vi "TLB Native Dynamic Events ver 0.26c.vi"() -> ()   [LabVIEW 2018] (continued)
                  tunnel: [w1148 w1154] -> w1144
                  tunnel: w1136 -> [w1146 w1152]
                  frame False {
                    n432 = for {
                      tunnel: string[] ["START TIMER", "OPEN CLAW", ""] ("element") -> [w1149] mode=indexing
                      shift-right: [w1151] -> w1148
                      shift-left: w1146 -> [w1150]
                      n433 = Enqueue Element(queue=w1150, element=w1149) -> (queue out=w1151:refnum<queue>)  [unwired: 2 in, 2 out]
                    }
                  }
                  frame True {
                    n434 = for {
                      shift-right: [w1156] -> w1154
                      shift-left: w1152 -> [w1157]
                      tunnel: string[] ["CAM CLOSE", "", ""] -> [w1155] mode=indexing
                      n435 = Enqueue Element(queue=w1157, element=w1155) -> (queue out=w1156:refnum<queue>)  [unwired: 2 in, 2 out]
                    }
                  }
                }
                n436 = Or(x=w1135, y=w1140) -> (x .or. y?=w1142:bool)
                n437 = Select(t=State_Type_Definitions,_for_0.26g_versions_and_later_2."True Stop" ("Enum"), s=w1140, f=State_Type_Definitions,_for_0.26g_versions_and_later_2."True Stop" ("Enum")) -> (s? t:f=w1137:T18)
                n438 = Select(t=w1137, s=w1142, f=State_Type_Definitions,_for_0.26g_versions_and_later_2."Task 5D" ("Enum")) -> (s? t:f=w1141:T18)
              }
              frame "Exit" {
                n439 = for {
                  shift-right: [w1164] -> w1161
                  shift-left: w1158 -> [w1165]
                  tunnel: string[] ["STOP", "RESET ENCODERS", "RESET YAW", "ARDUINO MODE 0"] -> [w1163] mode=indexing
                  n440 = Enqueue Element(queue=w1165, element=w1163) -> (queue out=w1164:refnum<queue>)  [unwired: 2 in, 2 out]
                }
              }
            }
          }
          frame 20 {
            # ">>> yStepper command>>>"
            n441 = Dequeue Element(queue=w1179, timeout in ms (-1)=w1180, error in (no error)=w1181) -> (element=w1183:T10)  [unwired: 3 out]
            n442 = formula code="if (pos < 100)\ny = 41;\n\nelse if (pos >= 100 && pos <= 140)\ny = 30;\n\nelse if (pos >= 141 && pos <= 170)\ny = 25;\n\nelse if (pos >= 171 &&pos <= 180) \ny = 20;\n\nelse if (pos >= 181&& pos <= 200)\ny = 15;\n\nelse if (pos >= 201 && pos <= 230)\ny = 10;\n\nelse if (pos >= 231 && pos <= 320)\ny = 8;\n\nelse if (pos > 320)\ny = 0;"("pos"=w1171) -> ("y"=w1174:dbl)
            n443 = To Unsigned Byte Integer(number=w1174) -> (unsigned 8bit integer=w1169:u8)
            n444 = Equal?(x=w1170, y=w1169) -> (x = y?=w1168:bool)
            n445 = case shown="\"Start Task 1\", Default" w1183 {
              tunnel: [w1190 State_Type_Definitions,_for_0.26g_versions_and_later_2."True Stop" ("Enum")] -> w1177
              tunnel: [w1193 w1210] -> w1175
              tunnel: [State_Type_Definitions,_for_0.26g_versions_and_later_2."Idle" ("Enum") State_Type_Definitions,_for_0.26g_versions_and_later_2."Shutdown" ("Enum")] -> w1176
              tunnel: w1182 -> [w1189 _]
              tunnel: w1178 -> [w1185 w1207]
              tunnel: w1168 -> [w1184 _]
              frame "Start Task 1", Default {
                # ">> T: Breaks out of state loop; F: Stays in loop>>"
                # ">> Manual override >>"
                # ">> Checks if time is up>>"
                # "Stays in Task 5D until the object is detected"
                # "T: Go back to idle, F: Continue with task\""
                # ">> Manual override >>"
                n446 = case shown="False" w1184 {
                  tunnel: [w1197 w1203] -> w1193
                  tunnel: w1185 -> [w1195 w1201]
                  frame False {
                    n447 = for {
                      tunnel: string[] ["READ STEPPER VALUES", "Y STEPPER CONTROL", ""] ("element") -> [w1198] mode=indexing
                      shift-right: [w1200] -> w1197
                      shift-left: w1195 -> [w1199]
                      n448 = Enqueue Element(queue=w1199, element=w1198) -> (queue out=w1200:refnum<queue>)  [unwired: 2 in, 2 out]
                    }
                  }
                  frame True {
                    n449 = for {
                      shift-right: [w1205] -> w1203
                      shift-left: w1201 -> [w1206]
                      tunnel: string[] ["CAM CLOSE", "DISPOSE BUFFERS", ""] -> [w1204] mode=indexing
                      n450 = Enqueue Element(queue=w1206, element=w1204) -> (queue out=w1205:refnum<queue>)  [unwired: 2 in, 2 out]
                    }
                  }
                }
                n451 = Or(x=w1184, y=w1189) -> (x .or. y?=w1191:bool)
                n452 = Select(t=State_Type_Definitions,_for_0.26g_versions_and_later_2."True Stop" ("Enum"), s=w1189, f=State_Type_Definitions,_for_0.26g_versions_and_later_2."Task 5F: ARM GRAB HEIGHT" ("Enum")) -> (s? t:f=w1186:T18)
                n453 = Select(t=w1186, s=w1191, f=State_Type_Definitions,_for_0.26g_versions_and_later_2."Task 5E: POSITION ARM" ("Enum")) -> (s? t:f=w1190:T18)
              }
              frame "Exit" {
                n454 = for {
                  shift-right: [w1213] -> w1210
                  shift-left: w1207 -> [w1214]
                  tunnel: string[] ["STOP", "RESET ENCODERS", "RESET YAW", "ARDUINO MODE 0"] -> [w1212] mode=indexing
                  n455 = Enqueue Element(queue=w1214, element=w1212) -> (queue out=w1213:refnum<queue>)  [unwired: 2 in, 2 out]
                }
              }
            }
            n456 = Bundle By Name(cluster=w1173, "yStepper desired"=w1169) -> (w1172:T20)
          }
          frame 21 {
            # ">>> Motor control cluster >>>"
            # ">>> yStepper command>>>"
            # ">> Manual override >>"
            n457 = Dequeue Element(queue=w1225, timeout in ms (-1)=w1224, error in (no error)=w1226) -> (element=w1223:T10)  [unwired: 3 out]
            n458 = Equal?(x=w1222, y=u8 1) -> (x = y?=w1220:bool)
            n459 = case shown="\"Start Task 1\", Default" w1223 {
              tunnel: [w1236 State_Type_Definitions,_for_0.26g_versions_and_later_2."True Stop" ("Enum")] -> w1227
              tunnel: [w1239 w1256] -> w1228
              tunnel: [State_Type_Definitions,_for_0.26g_versions_and_later_2."Idle" ("Enum") State_Type_Definitions,_for_0.26g_versions_and_later_2."Shutdown" ("Enum")] -> w1229
              tunnel: w1220 -> [w1235 _]
              tunnel: w1219 -> [w1234 _]
              tunnel: w1218 -> [w1230 w1253]
              frame "Start Task 1", Default {
                # "Stays in Task 5F until stepper reaches desired \nheight"
                # "T: Go back to idle, F: Continue with task\""
                # ">> Manual override >>"
                n460 = case shown="True" w1235 {
                  tunnel: [w1243 w1249] -> w1239
                  tunnel: w1230 -> [w1241 w1247]
                  frame False {
                    n461 = for {
                      tunnel: string[] ["Z STEPPER GRAB HEIGHT", "READ STEPPER VALUES"] ("element") -> [w1244] mode=indexing
                      shift-right: [w1246] -> w1243
                      shift-left: w1241 -> [w1245]
                      n462 = Enqueue Element(queue=w1245, element=w1244) -> (queue out=w1246:refnum<queue>)  [unwired: 2 in, 2 out]
                    }
                  }
                  frame True {
                    n463 = for {
                      shift-right: [w1251] -> w1249
                      shift-left: w1247 -> [w1252]
                      tunnel: string[] ["SET TIMER 5", "CLOSE CLAW", ""] -> [w1250] mode=indexing
                      n464 = Enqueue Element(queue=w1252, element=w1250) -> (queue out=w1251:refnum<queue>)  [unwired: 2 in, 2 out]
                    }
                  }
                }
                n465 = Or(x=w1235, y=w1234) -> (x .or. y?=w1237:bool)
                n466 = Select(t=State_Type_Definitions,_for_0.26g_versions_and_later_2."True Stop" ("Enum"), s=w1234, f=State_Type_Definitions,_for_0.26g_versions_and_later_2."Task 5G: CLOSE CLAW" ("Enum")) -> (s? t:f=w1231:T18)
                n467 = Select(t=w1231, s=w1237, f=State_Type_Definitions,_for_0.26g_versions_and_later_2."Task 5F: ARM GRAB HEIGHT" ("Enum")) -> (s? t:f=w1236:T18)
              }
              frame "Exit" {
                n468 = for {
                  shift-right: [w1259] -> w1256
                  shift-left: w1253 -> [w1260]
                  tunnel: string[] ["STOP", "RESET ENCODERS", "RESET YAW", "ARDUINO MODE 0"] -> [w1258] mode=indexing
                  n469 = Enqueue Element(queue=w1260, element=w1258) -> (queue out=w1259:refnum<queue>)  [unwired: 2 in, 2 out]
                }
              }
            }
          }
          frame 22 {
            # ">>> yStepper command>>>"
            # ">> Manual override >>"
            n470 = Dequeue Element(queue=w1271, timeout in ms (-1)=w1270, error in (no error)=w1269) -> (element=w1268:T10)  [unwired: 3 out]
            n471 = case shown="\"Start Task 1\", Default" w1268 {
              tunnel: [w1280 State_Type_Definitions,_for_0.26g_versions_and_later_2."True Stop" ("Enum")] -> w1273
              tunnel: [w1283 w1300] -> w1266
              tunnel: [State_Type_Definitions,_for_0.26g_versions_and_later_2."Idle" ("Enum") State_Type_Definitions,_for_0.26g_versions_and_later_2."Shutdown" ("Enum")] -> w1265
              tunnel: w1267 -> [w1274 _]
              tunnel: w1272 -> [w1279 w1297]
              tunnel: w1263 -> [w1278 _]
              frame "Start Task 1", Default {
                # ">> Is time up? >>"
                # "Determines if object is in range to pick up"
                # ">> Manual override >>"
                n472 = case shown="True" w1278 {
                  tunnel: [w1287 w1293] -> w1283
                  tunnel: w1279 -> [w1285 w1291]
                  frame False {
                    n473 = for {
                      tunnel: string[] ["CLOSE CLAW", "START TIMER"] ("element") -> [w1288] mode=indexing
                      shift-right: [w1290] -> w1287
                      shift-left: w1285 -> [w1289]
                      n474 = Enqueue Element(queue=w1289, element=w1288) -> (queue out=w1290:refnum<queue>)  [unwired: 2 in, 2 out]
                    }
                  }
                  frame True {
                    n475 = for {
                      shift-right: [w1295] -> w1293
                      shift-left: w1291 -> [w1296]
                      tunnel: string[] ["READ STEPPER VALUES", "", ""] -> [w1294] mode=indexing
                      n476 = Enqueue Element(queue=w1296, element=w1294) -> (queue out=w1295:refnum<queue>)  [unwired: 2 in, 2 out]
                    }
                  }
                }
                n477 = Or(x=w1278, y=w1274) -> (x .or. y?=w1281:bool)
                n478 = Select(t=State_Type_Definitions,_for_0.26g_versions_and_later_2."True Stop" ("Enum"), s=w1274, f=State_Type_Definitions,_for_0.26g_versions_and_later_2."Task 5H: RAISE ARM" ("Enum")) -> (s? t:f=w1276:T18)
                n479 = Select(t=w1276, s=w1281, f=State_Type_Definitions,_for_0.26g_versions_and_later_2."Task 5G: CLOSE CLAW" ("Enum")) -> (s? t:f=w1280:T18)
              }
              frame "Exit" {
                n480 = for {
                  shift-right: [w1303] -> w1300
                  shift-left: w1297 -> [w1304]
                  tunnel: string[] ["STOP", "RESET ENCODERS", "RESET YAW", "ARDUINO MODE 0"] -> [w1302] mode=indexing
                  n481 = Enqueue Element(queue=w1304, element=w1302) -> (queue out=w1303:refnum<queue>)  [unwired: 2 in, 2 out]
                }
              }
            }
          }
          frame 23 {
            # ">>> yStepper command>>>"
            # ">> Manual override >>"
            n482 = Dequeue Element(queue=w1315, timeout in ms (-1)=w1314, error in (no error)=w1316) -> (element=w1313:T10)  [unwired: 3 out]
            n483 = Equal?(x=w1312, y=u8 60) -> (x = y?=w1310:bool)
            n484 = case shown="\"Start Task 1\", Default" w1313 {
              tunnel: [w1326 State_Type_Definitions,_for_0.26g_versions_and_later_2."True Stop" ("Enum")] -> w1317
              tunnel: [w1329 w1346] -> w1318
              tunnel: [State_Type_Definitions,_for_0.26g_versions_and_later_2."Idle" ("Enum") State_Type_Definitions,_for_0.26g_versions_and_later_2."Shutdown" ("Enum")] -> w1319
              tunnel: w1310 -> [w1325 _]
              tunnel: w1309 -> [w1324 _]
              tunnel: w1308 -> [w1320 w1343]
              frame "Start Task 1", Default {
                # "Stays in Task 5_A until stepper reaches desired \nheight"
                # "T: Go back to idle, F: Continue with task\""
                # ">> Manual override >>"
                n485 = case shown="False" w1325 {
                  tunnel: [w1333 w1339] -> w1329
                  tunnel: w1320 -> [w1331 w1337]
                  frame False {
                    n486 = for {
                      tunnel: string[] ["Z STEPPER CAM HEIGHT", "READ STEPPER VALUES"] ("element") -> [w1334] mode=indexing
                      shift-right: [w1336] -> w1333
                      shift-left: w1331 -> [w1335]
                      n487 = Enqueue Element(queue=w1335, element=w1334) -> (queue out=w1336:refnum<queue>)  [unwired: 2 in, 2 out]
                    }
                  }
                  frame True {
                    n488 = for {
                      shift-right: [w1341] -> w1339
                      shift-left: w1337 -> [w1342]
                      tunnel: string[] ["ARDUINO - ULTRASONIC", "READ ULTRASONIC", ""] -> [w1340] mode=indexing
                      n489 = Enqueue Element(queue=w1342, element=w1340) -> (queue out=w1341:refnum<queue>)  [unwired: 2 in, 2 out]
                    }
                  }
                }
                n490 = Or(x=w1325, y=w1324) -> (x .or. y?=w1327:bool)
                n491 = Select(t=State_Type_Definitions,_for_0.26g_versions_and_later_2."True Stop" ("Enum"), s=w1324, f=State_Type_Definitions,_for_0.26g_versions_and_later_2."True Stop" ("Enum")) -> (s? t:f=w1321:T18)
                n492 = Select(t=w1321, s=w1327, f=State_Type_Definitions,_for_0.26g_versions_and_later_2."Task 5H: RAISE ARM" ("Enum")) -> (s? t:f=w1326:T18)
              }
              frame "Exit" {
                n493 = for {
                  shift-right: [w1349] -> w1346
                  shift-left: w1343 -> [w1350]
                  tunnel: string[] ["STOP", "RESET ENCODERS", "RESET YAW", "ARDUINO MODE 0"] -> [w1348] mode=indexing
                  n494 = Enqueue Element(queue=w1350, element=w1348) -> (queue out=w1349:refnum<queue>)  [unwired: 2 in, 2 out]
                }
              }
            }
          }
          frame 24 {
            # ">>> yStepper command>>>"
            n495 = Dequeue Element(queue=w1360, timeout in ms (-1)=w1359, error in (no error)=w1358) -> (element=w1365:T10)  [unwired: 3 out]
            n496 = Equal?(x=w1356, y=u8 60) -> (x = y?=w1355:bool)
            n497 = case shown="\"Start Task 1\", Default" w1365 {
              tunnel: [w1372 State_Type_Definitions,_for_0.26g_versions_and_later_2."True Stop" ("Enum")] -> w1363
              tunnel: [w1371 w1389] -> w1362
              tunnel: [State_Type_Definitions,_for_0.26g_versions_and_later_2."Idle" ("Enum") State_Type_Definitions,_for_0.26g_versions_and_later_2."Shutdown" ("Enum")] -> w1364
              tunnel: w1361 -> [w1367 _]
              tunnel: w1357 -> [w1369 _]
              tunnel: w1355 -> [w1366 _]
              frame "Start Task 1", Default {
                n498 = case shown="False" w1366 {
                  tunnel: [w1377 w1383] -> w1371
                  tunnel: w1369 -> [w1375 w1381]
                  frame False {
                    n499 = for {
                      tunnel: string[] ["Z STEPPER CAM HEIGHT", "READ STEPPER VALUES"] ("element") -> [w1378] mode=indexing
                      shift-right: [w1380] -> w1377
                      shift-left: w1375 -> [w1379]
                      n500 = Enqueue Element(queue=w1379, element=w1378) -> (queue out=w1380:refnum<queue>)  [unwired: 2 in, 2 out]
                    }
                  }
                  frame True {
                    n501 = for {
                      shift-right: [w1385] -> w1383
                      shift-left: w1381 -> [w1386]
                      tunnel: string[] ["CAM ACQ", "OPEN LOG CAM"] -> [w1384] mode=indexing
                      n502 = Enqueue Element(queue=w1386, element=w1384) -> (queue out=w1385:refnum<queue>)  [unwired: 2 in, 2 out]
                    }
                  }
                }
                n503 = Or(x=w1366, y=w1367) -> (x .or. y?=w1368:bool)
                n504 = Select(t=State_Type_Definitions,_for_0.26g_versions_and_later_2."Task 6_B" ("Enum"), s=w1368, f=State_Type_Definitions,_for_0.26g_versions_and_later_2."Task 6_A" ("Enum")) -> (s? t:f=w1372:T18)
              }
              frame "Exit" {
                n505 = for {
                  shift-right: [w1392] -> w1389
                  shift-left: _ -> [w1393]
                  tunnel: string[] ["STOP", "RESET ENCODERS", "RESET YAW", "ARDUINO MODE 0"] -> [w1391] mode=indexing
                  n506 = Enqueue Element(queue=w1393, element=w1391) -> (queue out=w1392:refnum<queue>)  [unwired: 2 in, 2 out]
                }
              }
            }
          }
          frame 25 {
            # ">>> yStepper command>>>"
            n507 = Dequeue Element(queue=w1405, timeout in ms (-1)=w1403, error in (no error)=w1404) -> (element=w1402:T10)  [unwired: 3 out]
            n508 = case shown="\"Start Task 1\", Default" w1402 {
              tunnel: [w1412 State_Type_Definitions,_for_0.26g_versions_and_later_2."True Stop" ("Enum")] -> w1398
              tunnel: [w1411 w1430] -> w1406
              tunnel: [State_Type_Definitions,_for_0.26g_versions_and_later_2."Idle" ("Enum") State_Type_Definitions,_for_0.26g_versions_and_later_2."Shutdown" ("Enum")] -> w1399
              tunnel: w1401 -> [w1407 _]
              tunnel: w1400 -> [w1409 _]
              tunnel: w1397 -> [w1408 w1427]
              frame "Start Task 1", Default {
                # ">> Manual override >>"
                n509 = case shown="False" w1409 {
                  tunnel: [w1417 w1423] -> w1411
                  tunnel: w1408 -> [w1416 w1421]
                  frame False {
                    n510 = for {
                      shift-right: [w1420] -> w1417
                      shift-left: w1416 -> [w1419]
                      tunnel: string[] ["CAM ACQ", "PROCESS IMAGE", "OPEN CLAW"] -> [w1418] mode=indexing
                      n511 = Enqueue Element(queue=w1419, element=w1418) -> (queue out=w1420:refnum<queue>)  [unwired: 2 in, 2 out]
                    }
                  }
                  frame True {
                    n512 = for {
                      shift-right: [w1425] -> w1423
                      shift-left: w1421 -> [w1426]
                      tunnel: string[] ["CAM ACQ", "PROCESS IMAGE", "CLOSE CLAW"] -> [w1424] mode=indexing
                      n513 = Enqueue Element(queue=w1426, element=w1424) -> (queue out=w1425:refnum<queue>)  [unwired: 2 in, 2 out]
                    }
                  }
                }
                n514 = Select(t=State_Type_Definitions,_for_0.26g_versions_and_later_2."True Stop" ("Enum"), s=w1407, f=State_Type_Definitions,_for_0.26g_versions_and_later_2."Task 6_B" ("Enum")) -> (s? t:f=w1412:T18)
              }
              frame "Exit" {
                # ">> State after true stop >>"
                # ">> Goes to true stop >>"
                n515 = for {
                  shift-right: [w1433] -> w1430
                  shift-left: w1427 -> [w1434]
                  tunnel: string[] ["STOP", "RESET ENCODERS", "RESET YAW", ""] -> [w1432] mode=indexing
                  n516 = Enqueue Element(queue=w1434, element=w1432) -> (queue out=w1433:refnum<queue>)  [unwired: 2 in, 2 out]
                }
              }
            }
          }
          frame 26 {
          }
          frame 27 {
            # ">>> Motor control cluster >>>"
            # ">>> yStepper command>>>"
            # ">> Manual override >>"
            n517 = Dequeue Element(queue=w1451, timeout in ms (-1)=w1450, error in (no error)=w1452) -> (element=w1449:T10)  [unwired: 3 out]
            n518 = Equal?(x=w1448, y=u8 60) -> (x = y?=w1446:bool)
            n519 = case shown="\"Start Task 1\", Default" w1449 {
              tunnel: [w1462 State_Type_Definitions,_for_0.26g_versions_and_later_2."True Stop" ("Enum")] -> w1453
              tunnel: [w1465 w1482] -> w1454
              tunnel: [State_Type_Definitions,_for_0.26g_versions_and_later_2."Idle" ("Enum") State_Type_Definitions,_for_0.26g_versions_and_later_2."Shutdown" ("Enum")] -> w1455
              tunnel: w1446 -> [w1461 _]
              tunnel: w1445 -> [w1460 _]
              tunnel: w1444 -> [w1456 w1479]
              frame "Start Task 1", Default {
                # "Stays in Task 5_A until stepper reaches desired \nheight"
                # "T: Go back to idle, F: Continue with task\""
                # ">> Manual override >>"
                n520 = case shown="False" w1461 {
                  tunnel: [w1469 w1475] -> w1465
                  tunnel: w1456 -> [w1467 w1473]
                  frame False {
                    n521 = for {
                      tunnel: string[] ["Z STEPPER CAM HEIGHT", "READ STEPPER VALUES"] ("element") -> [w1470] mode=indexing
                      shift-right: [w1472] -> w1469
                      shift-left: w1467 -> [w1471]
                      n522 = Enqueue Element(queue=w1471, element=w1470) -> (queue out=w1472:refnum<queue>)  [unwired: 2 in, 2 out]
                    }
                  }
                  frame True {
                    n523 = for {
                      shift-right: [w1477] -> w1475
                      shift-left: w1473 -> [w1478]
                      tunnel: string[] ["ARDUINO - ULTRASONIC", "READ ULTRASONIC", ""] -> [w1476] mode=indexing
                      n524 = Enqueue Element(queue=w1478, element=w1476) -> (queue out=w1477:refnum<queue>)  [unwired: 2 in, 2 out]
                    }
                  }
                }
                n525 = Or(x=w1461, y=w1460) -> (x .or. y?=w1463:bool)
                n526 = Select(t=State_Type_Definitions,_for_0.26g_versions_and_later_2."True Stop" ("Enum"), s=w1460, f=State_Type_Definitions,_for_0.26g_versions_and_later_2."Task 8B: MOVE TO BOX" ("Enum")) -> (s? t:f=w1457:T18)
                n527 = Select(t=w1457, s=w1463, f=State_Type_Definitions,_for_0.26g_versions_and_later_2."Task 8A: RAISE ARM" ("Enum")) -> (s? t:f=w1462:T18)
              }
              frame "Exit" {
                n528 = for {
                  shift-right: [w1485] -> w1482
                  shift-left: w1479 -> [w1486]
                  tunnel: string[] ["STOP", "RESET ENCODERS", "RESET YAW", "ARDUINO MODE 0"] -> [w1484] mode=indexing
                  n529 = Enqueue Element(queue=w1486, element=w1484) -> (queue out=w1485:refnum<queue>)  [unwired: 2 in, 2 out]
                }
              }
            }
          }
          frame 28 {
            w1494 = u8 15 ("y")
            # ">>> yStepper command>>>"
            n530 = Less?(x=w1491, y=w1494) -> (x < y?=w1492:bool)
            n531 = Dequeue Element(queue=w1498, timeout in ms (-1)=w1497, error in (no error)=w1499) -> (element=w1496:T10)  [unwired: 3 out]
            n532 = Less?(x=w1490, y=w1494) -> (x < y?=w1493:bool)
            n533 = And(x=w1493, y=w1492) -> (x .and. y?=w1489:bool)
            n534 = case shown="\"Start Task 1\", Default" w1496 {
              tunnel: [w1511 State_Type_Definitions,_for_0.26g_versions_and_later_2."True Stop" ("Enum")] -> w1501
              tunnel: [w1514 w1531] -> w1500
              tunnel: [State_Type_Definitions,_for_0.26g_versions_and_later_2."Idle" ("Enum") State_Type_Definitions,_for_0.26g_versions_and_later_2."Shutdown" ("Enum")] -> w1502
              tunnel: w1504 -> [w1510 _]
              tunnel: w1503 -> [w1506 w1528]
              tunnel: w1489 -> [w1505 _]
              frame "Start Task 1", Default {
                # "Stays in Task 5_B to capture image over 5 seconds"
                # "T: Go back to idle, F: Continue with task\""
                # ">> Manual override >>"
                n535 = case shown="True" w1505 {
                  tunnel: [w1518 w1524] -> w1514
                  tunnel: w1506 -> [w1516 w1522]
                  frame False {
                    n536 = for {
                      tunnel: string[] ["FORWARD", "READ ULTRASONIC", "READ NAVX"] ("element") -> [w1519] mode=indexing
                      shift-right: [w1521] -> w1518
                      shift-left: w1516 -> [w1520]
                      n537 = Enqueue Element(queue=w1520, element=w1519) -> (queue out=w1521:refnum<queue>)  [unwired: 2 in, 2 out]
                    }
                  }
                  frame True {
                    n538 = for {
                      shift-right: [w1526] -> w1524
                      shift-left: w1522 -> [w1527]
                      tunnel: string[] ["STOP", "RESET ENCODERS", "OPEN LOG CAM", "SET TIMER 2", "OPEN IMAQ REF"] -> [w1525] mode=indexing
                      n539 = Enqueue Element(queue=w1527, element=w1525) -> (queue out=w1526:refnum<queue>)  [unwired: 2 in, 2 out]
                    }
                  }
                }
                n540 = Or(x=w1505, y=w1510) -> (x .or. y?=w1512:bool)
                n541 = Select(t=State_Type_Definitions,_for_0.26g_versions_and_later_2."True Stop" ("Enum"), s=w1510, f=State_Type_Definitions,_for_0.26g_versions_and_later_2."Task 8C: CAM BURST" ("Enum")) -> (s? t:f=w1507:T18)
                n542 = Select(t=w1507, s=w1512, f=State_Type_Definitions,_for_0.26g_versions_and_later_2."Task 8B: MOVE TO BOX" ("Enum")) -> (s? t:f=w1511:T18)
              }
              frame "Exit" {
                n543 = for {
                  shift-right: [w1534] -> w1531
                  shift-left: w1528 -> [w1535]
                  tunnel: string[] ["STOP", "RESET ENCODERS", "RESET YAW", "ARDUINO MODE 0"] -> [w1533] mode=indexing
                  n544 = Enqueue Element(queue=w1535, element=w1533) -> (queue out=w1534:refnum<queue>)  [unwired: 2 in, 2 out]
                }
              }
            }
          }
          frame 29 {
            # ">>> Motor control cluster >>>"
            # ">>> yStepper command>>>"
            # ">> Manual override >>"
            n545 = Dequeue Element(queue=w1546, timeout in ms (-1)=w1545, error in (no error)=w1544) -> (element=w1543:T10)  [unwired: 3 out]
            n546 = case shown="\"Start Task 1\", Default" w1543 {
              tunnel: [w1555 State_Type_Definitions,_for_0.26g_versions_and_later_2."True Stop" ("Enum")] -> w1548
              tunnel: [w1558 w1575] -> w1541
              tunnel: [State_Type_Definitions,_for_0.26g_versions_and_later_2."Idle" ("Enum") State_Type_Definitions,_for_0.26g_versions_and_later_2."Shutdown" ("Enum")] -> w1540
              tunnel: w1542 -> [w1549 _]
              tunnel: w1547 -> [w1554 w1572]
              tunnel: w1538 -> [w1553 _]
              frame "Start Task 1", Default {
                # ">> Is time up? >>"
                # "Determines if object is in range to pick up"
                # ">> Manual override >>"
                n547 = case shown="True" w1553 {
                  tunnel: [w1562 w1568] -> w1558
                  tunnel: w1554 -> [w1560 w1566]
                  frame False {
                    n548 = for {
                      tunnel: string[] ["CAM ACQ", "START TIMER"] ("element") -> [w1563] mode=indexing
                      shift-right: [w1565] -> w1562
                      shift-left: w1560 -> [w1564]
                      n549 = Enqueue Element(queue=w1564, element=w1563) -> (queue out=w1565:refnum<queue>)  [unwired: 2 in, 2 out]
                    }
                  }
                  frame True {
                    n550 = for {
                      shift-right: [w1570] -> w1568
                      shift-left: w1566 -> [w1571]
                      tunnel: string[] ["CAM CLOSE", "PROCESS IMAGE", "SET TIMER 5"] -> [w1569] mode=indexing
                      n551 = Enqueue Element(queue=w1571, element=w1569) -> (queue out=w1570:refnum<queue>)  [unwired: 2 in, 2 out]
                    }
                  }
                }
                n552 = Or(x=w1553, y=w1549) -> (x .or. y?=w1556:bool)
                n553 = Select(t=State_Type_Definitions,_for_0.26g_versions_and_later_2."True Stop" ("Enum"), s=w1549, f=State_Type_Definitions,_for_0.26g_versions_and_later_2."Task 8D: PROCESS IMAGE" ("Enum")) -> (s? t:f=w1551:T18)
                n554 = Select(t=w1551, s=w1556, f=State_Type_Definitions,_for_0.26g_versions_and_later_2."Task 8C: CAM BURST" ("Enum")) -> (s? t:f=w1555:T18)
              }
              frame "Exit" {
                n555 = for {
                  shift-right: [w1578] -> w1575
                  shift-left: w1572 -> [w1579]
                  tunnel: string[] ["STOP", "RESET ENCODERS", "RESET YAW", "ARDUINO MODE 0"] -> [w1577] mode=indexing
                  n556 = Enqueue Element(queue=w1579, element=w1577) -> (queue out=w1578:refnum<queue>)  [unwired: 2 in, 2 out]
                }
              }
            }
          }
          frame 30 {
            # ">>> yStepper command>>>"
            n557 = Dequeue Element(queue=w1587, timeout in ms (-1)=w1586, error in (no error)=w1585) -> (element=w1584:T10)  [unwired: 3 out]
            n558 = case shown="\"Start Task 1\", Default" w1584 {
              tunnel: [w1599 State_Type_Definitions,_for_0.26g_versions_and_later_2."True Stop" ("Enum")] -> w1591
              tunnel: [w1602 w1619] -> w1590
              tunnel: [State_Type_Definitions,_for_0.26g_versions_and_later_2."Idle" ("Enum") State_Type_Definitions,_for_0.26g_versions_and_later_2."Shutdown" ("Enum")] -> w1592
              tunnel: w1588 -> [w1598 _]
              tunnel: w1589 -> [w1594 w1616]
              tunnel: w1582 -> [w1593 _]
              frame "Start Task 1", Default {
                # ">> T: Breaks out of state loop; F: Stays in loop>>"
                # ">> Manual override >>"
                # ">> Checks if time is up>>"
                # "Stays in Task 5D until the object is detected"
                # "T: Go back to idle, F: Continue with task\""
                # ">> Manual override >>"
                n559 = case shown="False" w1593 {
                  tunnel: [w1606 w1612] -> w1602
                  tunnel: w1594 -> [w1604 w1610]
                  frame False {
                    n560 = for {
                      tunnel: string[] ["START TIMER", "PROCESS IMAGE", ""] ("element") -> [w1607] mode=indexing
                      shift-right: [w1609] -> w1606
                      shift-left: w1604 -> [w1608]
                      n561 = Enqueue Element(queue=w1608, element=w1607) -> (queue out=w1609:refnum<queue>)  [unwired: 2 in, 2 out]
                    }
                  }
                  frame True {
                    n562 = for {
                      shift-right: [w1614] -> w1612
                      shift-left: w1610 -> [w1615]
                      tunnel: string[] ["RESET ENCODERS", "", ""] -> [w1613] mode=indexing
                      n563 = Enqueue Element(queue=w1615, element=w1613) -> (queue out=w1614:refnum<queue>)  [unwired: 2 in, 2 out]
                    }
                  }
                }
                n564 = Or(x=w1593, y=w1598) -> (x .or. y?=w1600:bool)
                n565 = Select(t=State_Type_Definitions,_for_0.26g_versions_and_later_2."True Stop" ("Enum"), s=w1598, f=State_Type_Definitions,_for_0.26g_versions_and_later_2."Task 8E: ROBOT ADJUST" ("Enum")) -> (s? t:f=w1595:T18)
                n566 = Select(t=w1595, s=w1600, f=State_Type_Definitions,_for_0.26g_versions_and_later_2."Task 8D: PROCESS IMAGE" ("Enum")) -> (s? t:f=w1599:T18)
              }
              frame "Exit" {
                n567 = for {
                  shift-right: [w1622] -> w1619
                  shift-left: w1616 -> [w1623]
                  tunnel: string[] ["STOP", "RESET ENCODERS", "RESET YAW", "ARDUINO MODE 0"] -> [w1621] mode=indexing
                  n568 = Enqueue Element(queue=w1623, element=w1621) -> (queue out=w1622:refnum<queue>)  [unwired: 2 in, 2 out]
                }
              }
            }
          }
          frame 31 {
            # ">>> Motor control cluster >>>"
            # ">>> yStepper command>>>"
            n569 = Dequeue Element(queue=w1640, timeout in ms (-1)=w1639, error in (no error)=w1638) -> (element=w1637:T10)  [unwired: 3 out]
            n570 = Subtract(x=w1635, y=300.0) -> (x-y=w1633:dbl)
            n571 = formula code="if (error <= -61&&error > -300){\ndistance = -15;\nxSpeed = -30;\n}\n\nelse if (error <= -51 && error >= -60){\ndistance = -10;\nxSpeed = -30;\n}\n\nelse if (error >= -50 && error <= 50){\ndistance = 0;\nxSpeed = 0;\n}\n\nelse if (error >= 51 && error <= 80){\ndistance = 10;\nxSpeed = 30;\n}\n\nelse if (error >= 81 && error <= 100){\ndistance = 15;\nxSpeed = 30;\n}\n\nelse if (error >= 101 && error <= 120){\ndistance = 20;\nxSpeed = 30;\n}\n\nelse if (error >= 121 && error < 300){\ndistance = 25;\nxSpeed = 30;\n}\n\nelse{\ndistance = 0;\nxSpeed = 0;\n}"("error"=w1633) -> ("distance"=w1628:dbl, "xSpeed"=w1630:dbl)
            n572 = formula code="if (target > 0){\nif (current  >= target)\noutput = 1;\n\nelse if (current != target)\noutput = 0;\n}\n\nelse if (target == 0){\nif (current == target)\noutput = 1;\n\nelse if (current != target)\noutput = 0;\n}\n\nelse if (target < 0){\nif (current <= target)\noutput = 1;\n\nelse if (current != target)\noutput = 0;\n}\n\nelse if (current != target)\noutput = 0;"("target"=w1628, "current"=w1629) -> ("output"=w1627:dbl)
            n573 = Bundle By Name(cluster=w1632, "xSpeed"=w1630) -> (w1631:T19)
            n574 = Equal?(x=w1627, y=1.0) -> (x = y?=w1625:bool)
            n575 = case shown="\"Start Task 1\", Default" w1637 {
              tunnel: [w1652 State_Type_Definitions,_for_0.26g_versions_and_later_2."True Stop" ("Enum")] -> w1644
              tunnel: [w1655 w1672] -> w1643
              tunnel: [State_Type_Definitions,_for_0.26g_versions_and_later_2."Idle" ("Enum") State_Type_Definitions,_for_0.26g_versions_and_later_2."Shutdown" ("Enum")] -> w1645
              tunnel: w1641 -> [w1651 _]
              tunnel: w1642 -> [w1647 w1669]
              tunnel: w1625 -> [w1646 _]
              frame "Start Task 1", Default {
                # ">> T: Breaks out of state loop; F: Stays in loop>>"
                # ">> Manual override >>"
                # ">> Checks if time is up>>"
                # "Stays in Task 5D until the object is detected"
                # "T: Go back to idle, F: Continue with task\""
                # ">> Manual override >>"
                n576 = case shown="True" w1646 {
                  tunnel: [w1659 w1665] -> w1655
                  tunnel: w1647 -> [w1657 w1663]
                  frame False {
                    n577 = for {
                      tunnel: string[] ["X AXIS - SLOW", "READ ENCODERS", "READ NAVX"] ("element") -> [w1660] mode=indexing
                      shift-right: [w1662] -> w1659
                      shift-left: w1657 -> [w1661]
                      n578 = Enqueue Element(queue=w1661, element=w1660) -> (queue out=w1662:refnum<queue>)  [unwired: 2 in, 2 out]
                    }
                  }
                  frame True {
                    n579 = for {
                      shift-right: [w1667] -> w1665
                      shift-left: w1663 -> [w1668]
                      tunnel: string[] ["SET TIMER 2", "STOP", "READ STEPPER VALUES", ""] -> [w1666] mode=indexing
                      n580 = Enqueue Element(queue=w1668, element=w1666) -> (queue out=w1667:refnum<queue>)  [unwired: 2 in, 2 out]
                    }
                  }
                }
                n581 = Or(x=w1646, y=w1651) -> (x .or. y?=w1653:bool)
                n582 = Select(t=State_Type_Definitions,_for_0.26g_versions_and_later_2."True Stop" ("Enum"), s=w1651, f=State_Type_Definitions,_for_0.26g_versions_and_later_2."Task 8H: ARM ADJUST" ("Enum")) -> (s? t:f=w1648:T18)
                n583 = Select(t=w1648, s=w1653, f=State_Type_Definitions,_for_0.26g_versions_and_later_2."Task 8E: ROBOT ADJUST" ("Enum")) -> (s? t:f=w1652:T18)
              }
              frame "Exit" {
                n584 = for {
                  shift-right: [w1675] -> w1672
                  shift-left: w1669 -> [w1676]
                  tunnel: string[] ["STOP", "RESET ENCODERS", "RESET YAW", "ARDUINO MODE 0"] -> [w1674] mode=indexing
                  n585 = Enqueue Element(queue=w1676, element=w1674) -> (queue out=w1675:refnum<queue>)  [unwired: 2 in, 2 out]
                }
              }
            }
          }
          frame 32 {
            # ">>> Motor control cluster >>>"
            # ">>> yStepper command>>>"
            # ">> Manual override >>"
            n586 = Dequeue Element(queue=w1687, timeout in ms (-1)=w1686, error in (no error)=w1685) -> (element=w1684:T10)  [unwired: 3 out]
            n587 = case shown="\"Start Task 1\", Default" w1684 {
              tunnel: [w1696 State_Type_Definitions,_for_0.26g_versions_and_later_2."True Stop" ("Enum")] -> w1689
              tunnel: [w1699 w1716] -> w1682
              tunnel: [State_Type_Definitions,_for_0.26g_versions_and_later_2."Idle" ("Enum") State_Type_Definitions,_for_0.26g_versions_and_later_2."Shutdown" ("Enum")] -> w1681
              tunnel: w1683 -> [w1690 _]
              tunnel: w1688 -> [w1695 w1713]
              tunnel: w1679 -> [w1694 _]
              frame "Start Task 1", Default {
                # ">> Is time up? >>"
                # "Determines if object is in range to pick up"
                # ">> Manual override >>"
                n588 = case shown="False" w1694 {
                  tunnel: [w1703 w1709] -> w1699
                  tunnel: w1695 -> [w1701 w1707]
                  frame False {
                    n589 = for {
                      tunnel: string[] ["CAM ACQ", "START TIMER"] ("element") -> [w1704] mode=indexing
                      shift-right: [w1706] -> w1703
                      shift-left: w1701 -> [w1705]
                      n590 = Enqueue Element(queue=w1705, element=w1704) -> (queue out=w1706:refnum<queue>)  [unwired: 2 in, 2 out]
                    }
                  }
                  frame True {
                    n591 = for {
                      shift-right: [w1711] -> w1709
                      shift-left: w1707 -> [w1712]
                      tunnel: string[] ["CAM CLOSE", "PROCESS IMAGE", "SET TIMER 3"] -> [w1710] mode=indexing
                      n592 = Enqueue Element(queue=w1712, element=w1710) -> (queue out=w1711:refnum<queue>)  [unwired: 2 in, 2 out]
                    }
                  }
                }
                n593 = Or(x=w1694, y=w1690) -> (x .or. y?=w1697:bool)
                n594 = Select(t=State_Type_Definitions,_for_0.26g_versions_and_later_2."True Stop" ("Enum"), s=w1690, f=State_Type_Definitions,_for_0.26g_versions_and_later_2."Task 8G: PROCESS IMAGE 2" ("Enum")) -> (s? t:f=w1692:T18)
                n595 = Select(t=w1692, s=w1697, f=State_Type_Definitions,_for_0.26g_versions_and_later_2."Task 8F: CAM BURST 2" ("Enum")) -> (s? t:f=w1696:T18)
              }
              frame "Exit" {
                n596 = for {
                  shift-right: [w1719] -> w1716
                  shift-left: w1713 -> [w1720]
                  tunnel: string[] ["STOP", "RESET ENCODERS", "RESET YAW", "ARDUINO MODE 0"] -> [w1718] mode=indexing
                  n597 = Enqueue Element(queue=w1720, element=w1718) -> (queue out=w1719:refnum<queue>)  [unwired: 2 in, 2 out]
                }
              }
            }
          }
          frame 33 {
            # ">>> yStepper command>>>"
            n598 = Dequeue Element(queue=w1728, timeout in ms (-1)=w1727, error in (no error)=w1726) -> (element=w1725:T10)  [unwired: 3 out]
            n599 = case shown="\"Start Task 1\", Default" w1725 {
              tunnel: [w1740 State_Type_Definitions,_for_0.26g_versions_and_later_2."True Stop" ("Enum")] -> w1732
              tunnel: [w1743 w1760] -> w1731
              tunnel: [State_Type_Definitions,_for_0.26g_versions_and_later_2."Idle" ("Enum") State_Type_Definitions,_for_0.26g_versions_and_later_2."Shutdown" ("Enum")] -> w1733
              tunnel: w1729 -> [w1739 _]
              tunnel: w1730 -> [w1735 w1757]
              tunnel: w1723 -> [w1734 _]
              frame "Start Task 1", Default {
                # ">> T: Breaks out of state loop; F: Stays in loop>>"
                # ">> Manual override >>"
                # ">> Checks if time is up>>"
                # "Stays in Task 5D until the object is detected"
                # "T: Go back to idle, F: Continue with task\""
                # ">> Manual override >>"
                n600 = case shown="False" w1734 {
                  tunnel: [w1747 w1753] -> w1743
                  tunnel: w1735 -> [w1745 w1751]
                  frame False {
                    n601 = for {
                      tunnel: string[] ["START TIMER", "PROCESS IMAGE", ""] ("element") -> [w1748] mode=indexing
                      shift-right: [w1750] -> w1747
                      shift-left: w1745 -> [w1749]
                      n602 = Enqueue Element(queue=w1749, element=w1748) -> (queue out=w1750:refnum<queue>)  [unwired: 2 in, 2 out]
                    }
                  }
                  frame True {
                    n603 = for {
                      shift-right: [w1755] -> w1753
                      shift-left: w1751 -> [w1756]
                      tunnel: string[] ["READ STEPPER VALUES", "Y STEPPER CONTROL", ""] -> [w1754] mode=indexing
                      n604 = Enqueue Element(queue=w1756, element=w1754) -> (queue out=w1755:refnum<queue>)  [unwired: 2 in, 2 out]
                    }
                  }
                }
                n605 = Or(x=w1734, y=w1739) -> (x .or. y?=w1741:bool)
                n606 = Select(t=State_Type_Definitions,_for_0.26g_versions_and_later_2."True Stop" ("Enum"), s=w1739, f=State_Type_Definitions,_for_0.26g_versions_and_later_2."Task 8H: ARM ADJUST" ("Enum")) -> (s? t:f=w1736:T18)
                n607 = Select(t=w1736, s=w1741, f=State_Type_Definitions,_for_0.26g_versions_and_later_2."Task 8G: PROCESS IMAGE 2" ("Enum")) -> (s? t:f=w1740:T18)
              }
              frame "Exit" {
                n608 = for {
                  shift-right: [w1763] -> w1760
                  shift-left: w1757 -> [w1764]
                  tunnel: string[] ["STOP", "RESET ENCODERS", "RESET YAW", "ARDUINO MODE 0"] -> [w1762] mode=indexing
                  n609 = Enqueue Element(queue=w1764, element=w1762) -> (queue out=w1763:refnum<queue>)  [unwired: 2 in, 2 out]
                }
              }
            }
          }
          frame 34 {
            # ">>> yStepper command>>>"
            n610 = Dequeue Element(queue=w1778, timeout in ms (-1)=w1779, error in (no error)=w1780) -> (element=w1782:T10)  [unwired: 3 out]
            n611 = formula code="if (pos < 70)\ny = 43;\n\nelse if (pos >= 71 &&pos <= 80)\ny = 40;\n\nelse if (pos >= 81 && pos <= 90)\ny = 38;\n\nelse if (pos >= 91 &&pos <= 120)\ny = 35;\n\nelse if (pos >= 121 && pos <= 140)\ny = 30;\n\nelse if (pos >= 141 && pos <= 170)\ny = 26;\n\nelse if (pos >= 171 &&pos <= 220) \ny = 20;\n\nelse if (pos >= 221&& pos <= 240)\ny = 15;\n\nelse if (pos >= 241 && pos <= 250)\ny = 10;\n\nelse if (pos >= 251)\ny = 0;"("pos"=w1770) -> ("y"=w1773:dbl)
            n612 = To Unsigned Byte Integer(number=w1773) -> (unsigned 8bit integer=w1768:u8)
            n613 = Equal?(x=w1769, y=w1768) -> (x = y?=w1767:bool)
            n614 = case shown="\"Start Task 1\", Default" w1782 {
              tunnel: [w1789 State_Type_Definitions,_for_0.26g_versions_and_later_2."True Stop" ("Enum")] -> w1776
              tunnel: [w1792 w1809] -> w1774
              tunnel: [State_Type_Definitions,_for_0.26g_versions_and_later_2."Idle" ("Enum") State_Type_Definitions,_for_0.26g_versions_and_later_2."Shutdown" ("Enum")] -> w1775
              tunnel: w1781 -> [w1788 _]
              tunnel: w1777 -> [w1784 w1806]
              tunnel: w1767 -> [w1783 _]
              frame "Start Task 1", Default {
                # ">> T: Breaks out of state loop; F: Stays in loop>>"
                # ">> Manual override >>"
                # ">> Checks if time is up>>"
                # "Stays in Task 5D until the object is detected"
                # "T: Go back to idle, F: Continue with task\""
                # ">> Manual override >>"
                n615 = case shown="False" w1783 {
                  tunnel: [w1796 w1802] -> w1792
                  tunnel: w1784 -> [w1794 w1800]
                  frame False {
                    n616 = for {
                      tunnel: string[] ["READ STEPPER VALUES", "Y STEPPER CONTROL", ""] ("element") -> [w1797] mode=indexing
                      shift-right: [w1799] -> w1796
                      shift-left: w1794 -> [w1798]
                      n617 = Enqueue Element(queue=w1798, element=w1797) -> (queue out=w1799:refnum<queue>)  [unwired: 2 in, 2 out]
                    }
                  }
                  frame True {
                    n618 = for {
                      shift-right: [w1804] -> w1802
                      shift-left: w1800 -> [w1805]
                      tunnel: string[] ["DISPOSE BUFFERS", "READ STEPPER VALUES", ""] -> [w1803] mode=indexing
                      n619 = Enqueue Element(queue=w1805, element=w1803) -> (queue out=w1804:refnum<queue>)  [unwired: 2 in, 2 out]
                    }
                  }
                }
                n620 = Or(x=w1783, y=w1788) -> (x .or. y?=w1790:bool)
                n621 = Select(t=State_Type_Definitions,_for_0.26g_versions_and_later_2."True Stop" ("Enum"), s=w1788, f=State_Type_Definitions,_for_0.26g_versions_and_later_2."Task 8I: ARM GRAB HEIGHT" ("Enum")) -> (s? t:f=w1785:T18)
                n622 = Select(t=w1785, s=w1790, f=State_Type_Definitions,_for_0.26g_versions_and_later_2."Task 8H: ARM ADJUST" ("Enum")) -> (s? t:f=w1789:T18)
              }
              frame "Exit" {
                n623 = for {
                  shift-right: [w1812] -> w1809
                  shift-left: w1806 -> [w1813]
                  tunnel: string[] ["STOP", "RESET ENCODERS", "RESET YAW", "ARDUINO MODE 0"] -> [w1811] mode=indexing
                  n624 = Enqueue Element(queue=w1813, element=w1811) -> (queue out=w1812:refnum<queue>)  [unwired: 2 in, 2 out]
                }
              }
            }
            n625 = Bundle By Name(cluster=w1772, "yStepper desired"=w1768) -> (w1771:T20)
          }
          frame 35 {
            # ">>> Motor control cluster >>>"
            # ">>> yStepper command>>>"
            # ">> Manual override >>"
            n626 = Dequeue Element(queue=w1824, timeout in ms (-1)=w1823, error in (no error)=w1825) -> (element=w1822:T10)  [unwired: 3 out]
            n627 = Equal?(x=w1821, y=u8 1) -> (x = y?=w1819:bool)
            n628 = case shown="\"Start Task 1\", Default" w1822 {
              tunnel: [w1835 State_Type_Definitions,_for_0.26g_versions_and_later_2."True Stop" ("Enum")] -> w1826
              tunnel: [w1838 w1855] -> w1827
              tunnel: [State_Type_Definitions,_for_0.26g_versions_and_later_2."Idle" ("Enum") State_Type_Definitions,_for_0.26g_versions_and_later_2."Shutdown" ("Enum")] -> w1828
              tunnel: w1819 -> [w1834 _]
              tunnel: w1818 -> [w1833 _]
              tunnel: w1817 -> [w1829 w1852]
              frame "Start Task 1", Default {
                # "Stays in Task 5F until stepper reaches desired \nheight"
                # "T: Go back to idle, F: Continue with task\""
                # ">> Manual override >>"
                n629 = case shown="True" w1834 {
                  tunnel: [w1842 w1848] -> w1838
                  tunnel: w1829 -> [w1840 w1846]
                  frame False {
                    n630 = for {
                      tunnel: string[] ["Z STEPPER GRAB HEIGHT", "READ STEPPER VALUES"] ("element") -> [w1843] mode=indexing
                      shift-right: [w1845] -> w1842
                      shift-left: w1840 -> [w1844]
                      n631 = Enqueue Element(queue=w1844, element=w1843) -> (queue out=w1845:refnum<queue>)  [unwired: 2 in, 2 out]
                    }
                  }
                  frame True {
                    n632 = for {
                      shift-right: [w1850] -> w1848
                      shift-left: w1846 -> [w1851]
                      tunnel: string[] ["SET TIMER 2", "CLOSE CLAW", ""] -> [w1849] mode=indexing
                      n633 = Enqueue Element(queue=w1851, element=w1849) -> (queue out=w1850:refnum<queue>)  [unwired: 2 in, 2 out]
                    }
                  }
                }
                n634 = Or(x=w1834, y=w1833) -> (x .or. y?=w1836:bool)
                n635 = Select(t=State_Type_Definitions,_for_0.26g_versions_and_later_2."True Stop" ("Enum"), s=w1833, f=State_Type_Definitions,_for_0.26g_versions_and_later_2."Task 8J: CLOSE CLAW" ("Enum")) -> (s? t:f=w1830:T18)
                n636 = Select(t=w1830, s=w1836, f=State_Type_Definitions,_for_0.26g_versions_and_later_2."Task 8I: ARM GRAB HEIGHT" ("Enum")) -> (s? t:f=w1835:T18)
              }
              frame "Exit" {
                n637 = for {
                  shift-right: [w1858] -> w1855
                  shift-left: w1852 -> [w1859]
                  tunnel: string[] ["STOP", "RESET ENCODERS", "RESET YAW", "ARDUINO MODE 0"] -> [w1857] mode=indexing
                  n638 = Enqueue Element(queue=w1859, element=w1857) -> (queue out=w1858:refnum<queue>)  [unwired: 2 in, 2 out]
                }
              }
            }
          }
          frame 36 {
            # ">>> yStepper command>>>"
            # ">> Manual override >>"
            n639 = Dequeue Element(queue=w1870, timeout in ms (-1)=w1869, error in (no error)=w1868) -> (element=w1867:T10)  [unwired: 3 out]
            n640 = case shown="\"Start Task 1\", Default" w1867 {
              tunnel: [w1879 State_Type_Definitions,_for_0.26g_versions_and_later_2."True Stop" ("Enum")] -> w1872
              tunnel: [w1882 w1899] -> w1865
              tunnel: [State_Type_Definitions,_for_0.26g_versions_and_later_2."Idle" ("Enum") State_Type_Definitions,_for_0.26g_versions_and_later_2."Shutdown" ("Enum")] -> w1864
              tunnel: w1866 -> [w1873 _]
              tunnel: w1871 -> [w1878 w1896]
              tunnel: w1862 -> [w1877 _]
              frame "Start Task 1", Default {
                # ">> Is time up? >>"
                # "Determines if object is in range to pick up"
                # ">> Manual override >>"